vi "Main.vi"() -> ()   [LabVIEW 2020] (continued)
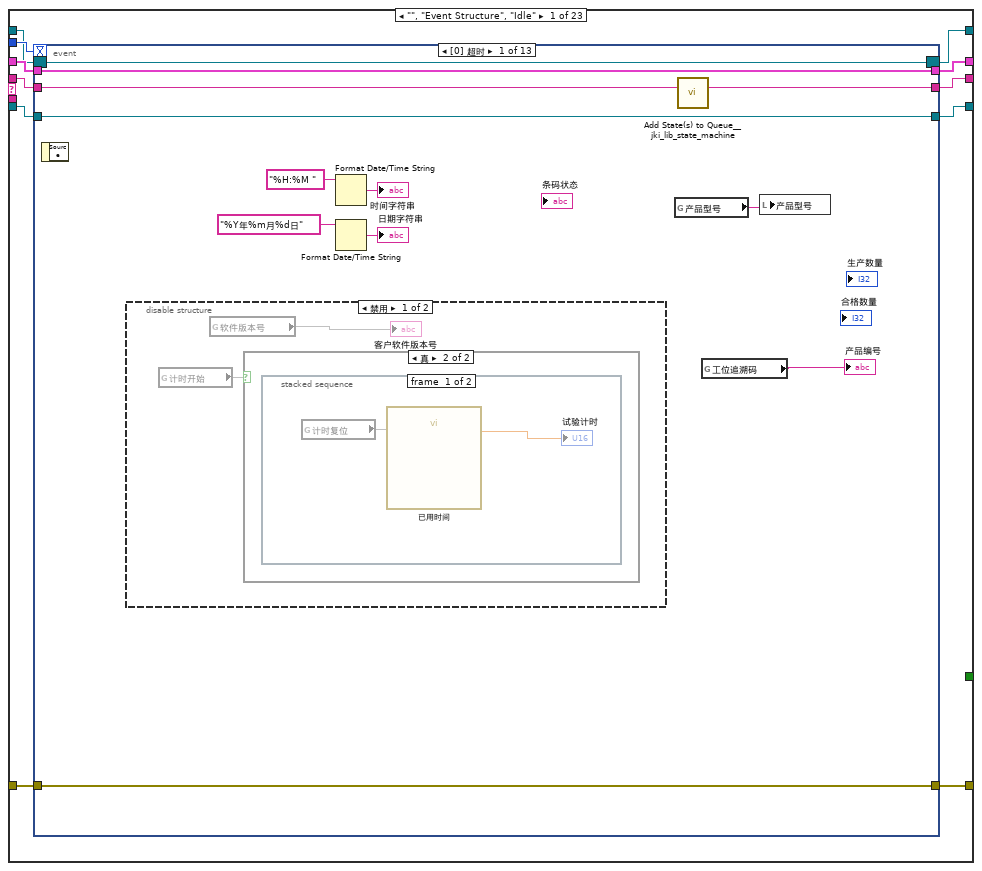
[diagram p2: hidden frame]
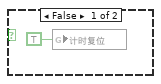
[diagram p3: hidden frame]
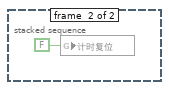
[diagram p4: hidden frame]
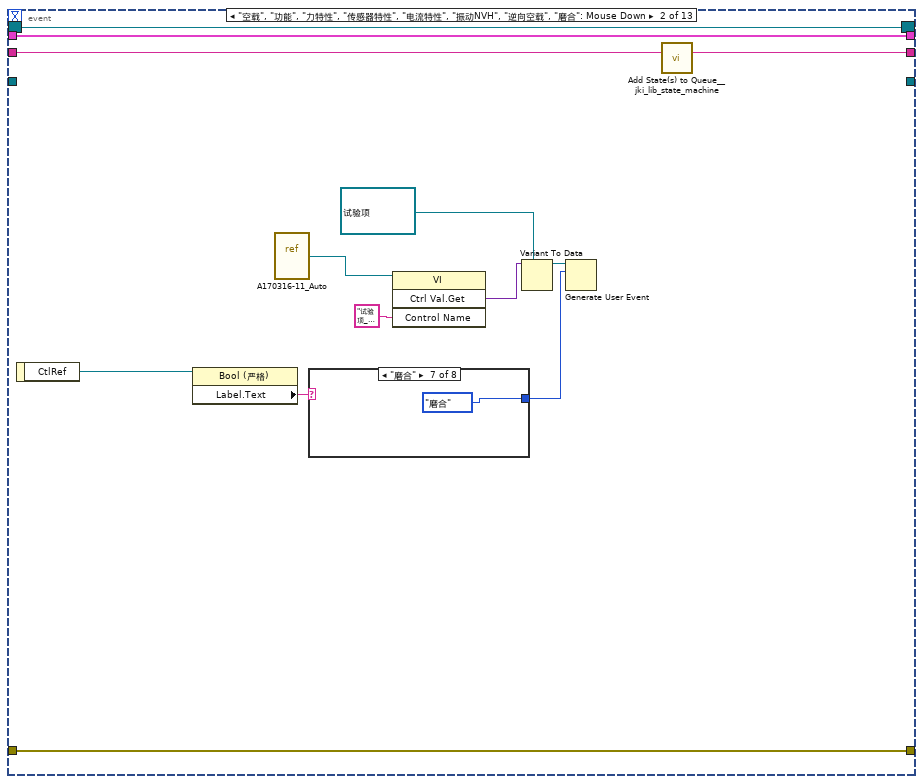
[diagram p6: hidden frame]
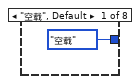
[diagram p7: hidden frame]
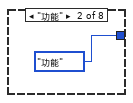
[diagram p8: hidden frame]
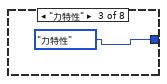
[diagram p9: hidden frame]
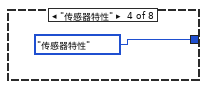
[diagram p10: hidden frame]
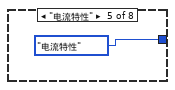
[diagram p11: hidden frame]
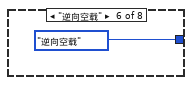
[diagram p12: hidden frame]
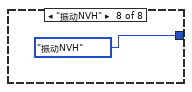
[diagram p13: hidden frame]
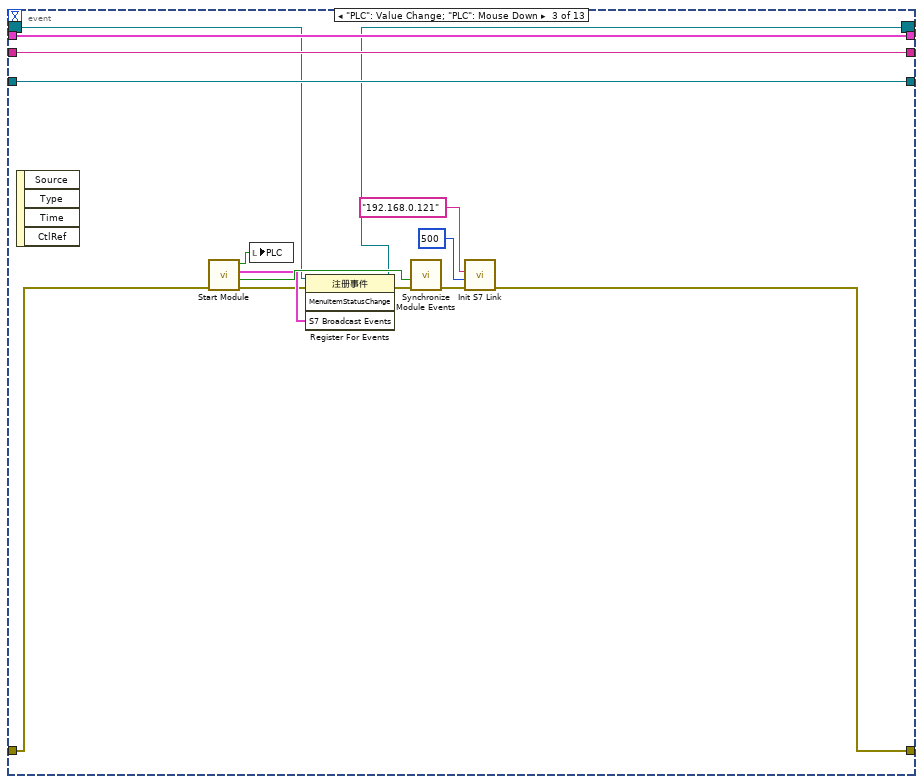
[diagram p14: hidden frame]
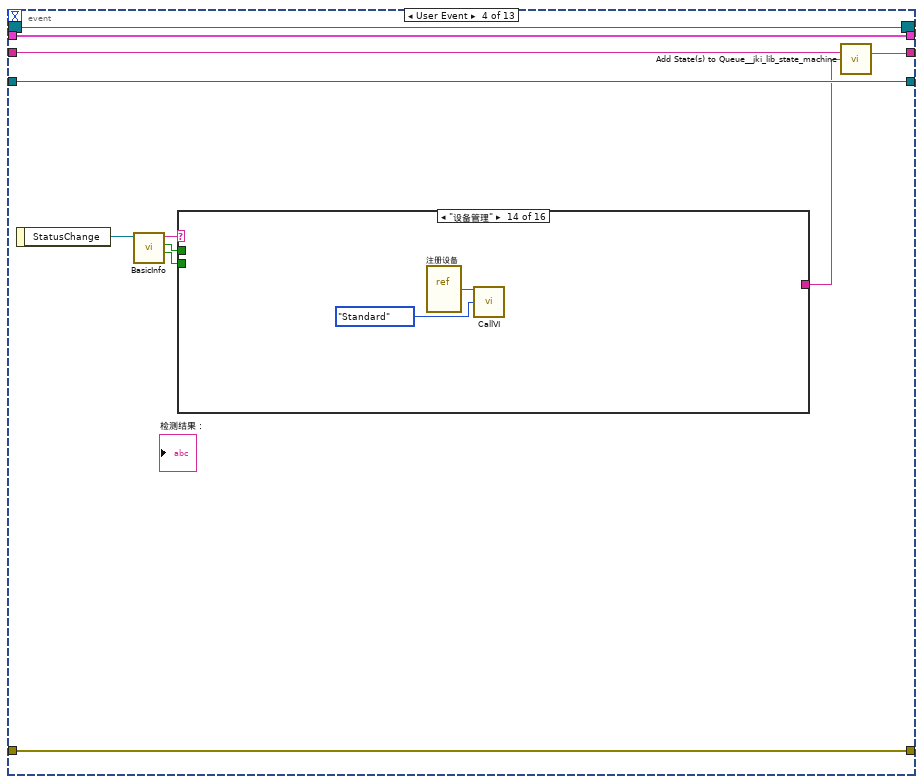
[diagram p15: hidden frame]
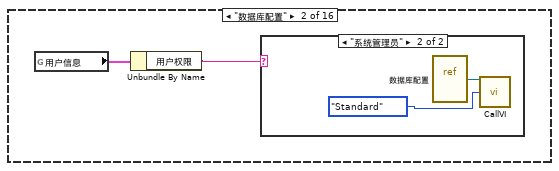
[diagram p17: hidden frame]
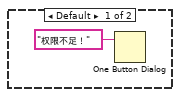
[diagram p18: hidden frame]
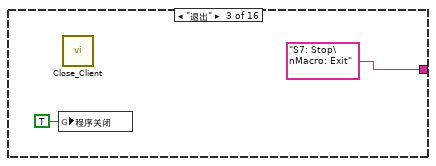
[diagram p19: hidden frame]
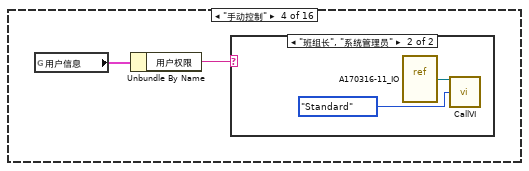
[diagram p20: hidden frame]
                  }
                }
              }
              frame True {
                n122 = Two Button Dialog(message="确定要退出自动？" ("消息")) -> (T button?=w202:bool)  [unwired: 2 in]
                n123 = case shown="真" w202 {
                  frame False {
                  }
                  frame True {
                    n124 = vi-ref "A170316-11_Auto.vi"() -> (w206:refnum<vi>)
                    n125 = invoke class="VI" method="Ctrl Val.Set"(reference=w206, "Control Name"="STEP" ("控件名"), "Value"="退出自动" ("控件名")) -> ()  [unwired: 2 in, 5 out]
                  }
                }
              }
            }
            n126 = call <vilib>:"Add State(s) to Queue__jki_lib_state_machine.vi"("State(s) in (\"\")"=w193) -> ("States Out"=w194:string)  [unwired: 14 in]
          }
          event "错误": Mouse Down {
            n127 = event-data() -> ()  [unwired: 1 in, 8 out]
            n128 = vi-ref "报警信息.vi"() -> (w209:refnum<vi>)
            n129 = call "CallVI.vi"("VI引用"=w209, "状态"=T3."Standard") -> ()  [unwired: 11 in, 3 out]
            n130 = call <vilib>:"Add State(s) to Queue__jki_lib_state_machine.vi"("State(s) in (\"\")"=w211) -> ("States Out"=w212:string)  [unwired: 14 in]
          }
          event Panel Close? {
            n131 = event-data() -> ()  [unwired: 1 in, 1 out]
            n132 = disable-structure shown="禁用" {
              frame Disabled {
                n133 = call "Close.vi"() -> ()  [unwired: 11 in, 1 out]
              }
              frame Enabled {
              }
            }
            n134 = global write "Global.vi" "程序关闭"(TRUE ("程序关闭")) -> ()
            n135 = call <vilib>:"Add State(s) to Queue__jki_lib_state_machine.vi"("State(s) in Front (\"\")"="S7: Stop\nMacro: Exit", "State(s) in (\"\")"=w221) -> ("States Out"=w220:string)  [unwired: 13 in]
            n136 = event-data("Discard?"=TRUE) -> ()  [unwired: 1 in, 1 out]
          }
          event "更换产品": Value Change {
            n137 = event-data() -> ("NewVal"=w224:refnum<vi>)  [unwired: 1 in, 5 out]
            n138 = stacked-sequence {
              tunnel: w224 -> [w230]
              tunnel: [w229] -> w222
              frame #0 {
                n139 = stacked-sequence {
                  tunnel: w230 -> [w231 _ _]
                  tunnel: [_ w242 _] -> w229
                  frame #0 {
                    n140 = disable-structure shown="禁用" {
                      frame Disabled {
                        n141 = vi-ref "Auto.vi"() -> (w238:refnum<vi>)
                        n142 = invoke class="VI" method="Ctrl Val.Get"(reference=w238, "Control Name"="产品_EVENT" ("控件名")) -> ("Get Control Value Variant"=w237:variant)  [unwired: 2 in, 3 out]
                        n143 = global read "Global.vi" "产品型号"() -> (w233:string)
                        n144 = local write "产品型号"(w233) -> ()
                        n145 = Variant To Data(type=refnum<user-event> refnum ("产品_EVENT"), Variant=w237) -> (data=w234:refnum<user-event>, error out=w232:errorcluster)  [unwired: 1 in]
                        n146 = Generate User Event(user event=w234, event data cluster=w233, error in=w232) -> ()  [unwired: 1 in, 2 out]
                      }
                      frame Enabled {
                      }
                    }
                    n147 = disable-structure shown="禁用" {
                      disable-tunnel: w231 -> [w240 _]
                      frame Disabled {
                        n148 = control-ref of="子面板"() -> (w239:refnum<vi>)
                        n149 = call "Call_SubPanal.vi"("VI引用句柄"=w240, "SubPnl引用句柄"=w239) -> ()  [unwired: 9 in, 1 out]
                      }
                      frame Enabled {
                      }
                    }
                  }
                  frame #1 {
                    n150 = global read "Global.vi" "启用CAN"() -> (w241:bool)
                    n151 = case shown="假" w241 {
                      tunnel: ["CAN: Stop" "CAN: Stop"] -> w242
                      frame False {
                      }
                      frame True {
                        (unwired) "CAN: Stop\nIdle\nCAN: Start"
                      }
                    }
                  }
                  frame #2 {
                    n152 = disable-structure shown="禁用" {
                      frame Disabled {
                        n153 = control-ref of="磨合"() -> (w245:refnum<vi>)
                        n154 = control-ref of="空载"() -> (w250:refnum<vi>)
                        n155 = control-ref of="功能"() -> (w251:refnum<vi>)
                        n156 = control-ref of="力特性"() -> (w252:refnum<vi>)
                        n157 = control-ref of="电流特性"() -> (w249:refnum<vi>)
                        n158 = control-ref of="传感器特性"() -> (w248:refnum<vi>)
                        n159 = control-ref of="逆向空载"() -> (w247:refnum<vi>)
                        n160 = control-ref of="振动NVH"() -> (w246:refnum<vi>)
                        n161 = global read "Global.vi" "试验项目"() -> (w255)
                        n162 = Build Array(w250, w251, w252, w249, w248, w247, w246, w245) -> (w254:refnum<vi>[])
                        n163 = for {
                          tunnel: w254 -> [w259] mode=indexing
                          tunnel: w255 -> [w260]
                          shift-right: [w256] -> _
                          shift-left: 2095 -> [w257]
                          i -> [w258]
                          n164 = case shown="真" w260 {
                            tunnel: w259 -> [w261 w269]
                            tunnel: w258 -> [_ _]
                            tunnel: w257 -> [w263 w266]
                            tunnel: [w263 w264] -> w256
                            frame False {
                              n165 = property class="Bool (严格)"(reference=w261, "Top"=2000) -> ()  [unwired: 1 in, 2 out]
                            }
                            frame True {
                              n166 = Add(x=w266, y=115) -> (x+y=w264:i32)
                              n167 = Bundle(w264, 1300) -> (w267:cluster{i32, i32})  [unwired: 1 in]
                              n168 = property class="Bool (严格)"(reference=w269, "Position"=w267) -> ()  [unwired: 1 in, 2 out]
                            }
                          }
                        }
                      }
                      frame Enabled {
                      }
                    }
                  }
                }
              }
            }
            n169 = call <vilib>:"Add State(s) to Queue__jki_lib_state_machine.vi"("State(s) in Front (\"\")"=w222, "State(s) in (\"\")"=w225) -> ("States Out"=w226:string)  [unwired: 13 in]
          }
          event "Andon": Value Change {
            w280 = "GP12终检" ("设备名称")
            n170 = event-data() -> ("NewVal"=w271:enum32{"未选择", "缺料报警", "质量报警", "故障报警"})  [unwired: 1 in]
            n171 = global read "Global1.vi" "用户信息"() -> (w270:T6)
            n172 = Unbundle By Name(w270) -> ("用户权限"=w279:string)
            n173 = case shown="\"故障报警\"" w271 {
              tunnel: w280 -> [_ _ _ _]
              tunnel: w279 -> [_ _ _ _]
              tunnel: [enum16{"设备离线", "设备正常", "设备缺料", "设备故障", "质量报警"}."设备正常" ("设备状态") enum16{"设备离线", "设备正常", "设备缺料", "设备故障", "质量报警"}."设备缺料" ("设备状态") enum16{"设备离线", "设备正常", "设备缺料", "设备故障", "质量报警"}."质量报警" ("设备状态") enum16{"设备离线", "设备正常", "设备缺料", "设备故障", "质量报警"}."设备故障" ("设备状态")] -> w277
              frame "未选择", Default {
              }
              frame "缺料报警" {
              }
              frame "质量报警" {
              }
              frame "故障报警" {
              }
            }
            n174 = Bundle By Name(cluster=T4 {"设备名称"="", "操作人员"="", "设备状态"=enum."设备离线", "附加信息"=""} ("设备信息"), "设备名称"=w280, "操作人员"=w279, "设备状态"=w277) -> (w272:T4)
            n175 = call "Change_Client.vi"("设备信息"=w272) -> ()  [unwired: 10 in, 1 out]
          }
        }
      }
      frame "---------- Core ----------" {
        n176 = call <vilib>:"Add State(s) to Queue__jki_lib_state_machine.vi"("State(s) in (\"\")"=w290) -> ("States Out"=w289:string)  [unwired: 14 in]
      }
      frame Default {
        w302 = 42 items=["No error", "Argument error", "Memory is full", "Out of zone", "End of file", "File already open", "Generic file I/O error", "File not found", "File permission error", "Disk is full", "Duplicate path", "Too many files open", "System feature not enabled", "Resource file not found", "Cannot add resource", "Resource not found", "Image not found", "Image memory error", "Pen does not exist", "Config type invalid", "Config token not found", "Config parse error", "Config memory error", "Bad external code format", "Bad external code offset", "External code not present", "Null window", "Destroy window error", "Null menu", "Print aborted", "Bad print record", "Print driver error", "Windows error during printing", "Memory error during printing", "Print dialog error", "Generic print error", "Invalid device refnum", "Device not found", "Device parameter error", "Device unit error", "Cannot open device", "Device call aborted", "Generic error", "Cancelled by user", "Object ID too low", "Object ID too high", "Object not in heap", "Unknown heap", "Unknown object (invalid DefProc)", "Unknown object (DefProc not in table)", "Message out of range", "Invalid (null) method", "Unknown message", "Manager call not supported", "Bad address", "Network operation in progress", "Network operation timed out", "Connection is busy", "Network attribute not supported", "Network error", "Address in use", "System out of memory", "Connection aborted", "Connection refused", "Not connected", "Already connected", "Connection closed", "Initialization error (interapplication manager)", "Bad occurrence", "Wait on unbound occurrence handler", "Occurrence queue overflow", "Datalog type conflict", "Unused", "Unrecognized type (interapplication manager)", "Memory corrupt", "Failed to make temporary DLL", "Old CIN version", "Drag socket not found", "Failed to load drop-object", "Failed to register OLE object", "Failed to release OLE object", "Format specifier type mismatch", "Unknown format specifier", "Too few format specifiers", "Too many format specifiers", "Scan failed", "Newer CIN version", "Error converting to variant", "Runtime menu error", "Password tampered", "Variant attribute not found", "Incompatible variant data type", "Event data is not available", "Event Store is not present", "Occurrence is not found", "Event Queue is not created", "Event info is not available", "Refnum passed is NULL", "Error retrieving Class GUID", "Error retrieving CoClass GUID", "Error retrieving TypeLib GUID.", "Bad built application magic bytes.", "Specific driver is different from the specific driver associated with the Logical Name.", "There is no session opened to the class driver.", "Max Error", "MAX - Error with config objects", "MAX - Error loading configuration", "MAX - Group not supported"]
        # "Current State"
        n177 = Format Into String(format string="Software Exception: Unhandled State \"%s\"." ("message"), error in=w298, w293) -> (resulting string=w301:string, error out=w300:errorcluster)  [unwired: 1 in]
        n178 = call <vilib>:"Error Cluster From Error Code.vi"("show call chain? (False)"=TRUE, "error in (no error)"=w300, "error message (\"\")"=w301, "error code (0)"=w302) -> ("error out"=w299:errorcluster)  [unwired: 5 in]
        n179 = call <vilib>:"Add State(s) to Queue__jki_lib_state_machine.vi"("State(s) in (\"\")"=w297) -> ("States Out"=w296:string)  [unwired: 14 in]
      }
      frame "Initialize Core Data" {
        # "originally closed?"
        # "exe?"
        n180 = property class="VI"() -> ("Front Panel.Open"=w313:bool)  [unwired: 2 in, 2 out]
        n181 = property class="App"() -> ("App.Kind"=w312:T5)  [unwired: 2 in, 2 out]
        n182 = control-ref of="Current VI Reference"() -> (w306:refnum<vi>)
        n183 = Not(x=w313) -> (.not. x?=w310:bool)
        n184 = Equal?(x=w312, y=T5."Run Time System" ("Application:Kind")) -> (x = y?=w309:bool)
        n185 = Or(x=w310, y=w309) -> (x .or. y?=w307:bool)
        n186 = Bundle By Name(cluster=w308, "Core.Current VI Reference"=w306, "Core.Close Panel on Exit?"=w307) -> (w315:T7)
        n187 = call <vilib>:"Add State(s) to Queue__jki_lib_state_machine.vi"("State(s) in (\"\")"=w317) -> ("States Out"=w316:string)  [unwired: 14 in]
      }
      frame "Error Handler" {
        n188 = call <vilib>:"General Error Handler.vi"("error in (no error)"=w321) -> ()  [unwired: 10 in, 5 out]
        n189 = call <vilib>:"Add State(s) to Queue__jki_lib_state_machine.vi"("State(s) in Front (\"\")"="/* Post Error States", "State(s) in (\"\")"=w325) -> ("States Out"=w324:string)  [unwired: 13 in]
      }
      frame "Exit" {
        n190 = Quit LabVIEW(quit? (T)=TRUE ("退出？(T)")) -> ()
        n191 = call <vilib>:"Add State(s) to Queue__jki_lib_state_machine.vi"("State(s) in (\"\")"=w333) -> ("States Out"=w332:string)  [unwired: 14 in]
      }
      frame "--------- Library --------" {
        n192 = call <vilib>:"Add State(s) to Queue__jki_lib_state_machine.vi"("State(s) in (\"\")"=w339) -> ("States Out"=w338:string)  [unwired: 14 in]
      }
      frame "S7: Initialize" {
        n193 = property on="PLC" class="Bool (严格)"("Val(Sgnl)"=FALSE ("值(信号)")) -> ()  [unwired: 2 in, 2 out]
      }
      frame "S7: Stop" {
        n194 = call "Stop Module.vi"("error in (no error)"=w348) -> ("error out"=w347:errorcluster)  [unwired: 10 in]
        n195 = call <vilib>:"Add State(s) to Queue__jki_lib_state_machine.vi"("State(s) in (\"\")"=w349) -> ("States Out"=w350:string)  [unwired: 14 in]
      }
      frame "CAN: Start" {
        n196 = call <vilib>:"Add State(s) to Queue__jki_lib_state_machine.vi"("State(s) in (\"\")"=w355) -> ("States Out"=w356:string)  [unwired: 14 in]
      }
      frame "CAN: Stop" {
        n197 = call <vilib>:"Add State(s) to Queue__jki_lib_state_machine.vi"("State(s) in (\"\")"=w361) -> ("States Out"=w362:string)  [unwired: 14 in]
      }
      frame "---------- Data ----------" {
        n198 = call <vilib>:"Add State(s) to Queue__jki_lib_state_machine.vi"("State(s) in (\"\")"=w370) -> ("States Out"=w369:string)  [unwired: 14 in]
      }
      frame "Data: Initialize" {
        (unwired) FALSE ("计时结束")
        w374 = T8 {"Current VI Reference"=refnum, "Close Panel on Exit?"=FALSE}  # Core
        w376 = TRUE  # Your Boolean data
        w375 = ""  # Your string data
        n199 = global write "Global.vi" "程序关闭"(FALSE ("程序关闭")) -> ()
        n200 = Bundle("Core"=w374, "Your Boolean data"=w376, "Your string data"=w375) -> (w378:T7)  [unwired: 1 in]
        n201 = call <vilib>:"Add State(s) to Queue__jki_lib_state_machine.vi"("State(s) in (\"\")"=w380) -> ("States Out"=w379:string)  [unwired: 14 in]
      }
      frame "Data: Cleanup" {
        n202 = Unbundle By Name(w383) -> ("Core.Current VI Reference"=w386:refnum<vi>)
        n203 = Close Reference(reference=w386, error in (no error)=w385) -> (error out=w384:errorcluster)
        n204 = call <vilib>:"Add State(s) to Queue__jki_lib_state_machine.vi"("State(s) in (\"\")"=w388) -> ("States Out"=w387:string)  [unwired: 14 in]
      }
      frame "---------- UI ----------" {
        # "Do not put any code in this frame.\n(It is a separator no-op. You can make a copy of this frame to create a new UI frame)"
        n205 = call <vilib>:"Add State(s) to Queue__jki_lib_state_machine.vi"("State(s) in (\"\")"=w394) -> ("States Out"=w393:string)  [unwired: 14 in]
      }
      frame "UI: Initialize" {
        n206 = disable-structure shown="启用" {
          disable-tunnel: [w408 _] -> w398
          disable-tunnel: w395 -> [w406 _]
          frame Enabled {
            n207 = vi-ref "A170316-11_Auto.vi"() -> (w407:refnum<vi>)
            n208 = property class="VI"(reference=w407) -> (reference out=w405:refnum<vi>, "FP.State"=w404:T3)  [unwired: 1 in, 1 out]
            n209 = case shown="\"Invalid\", \"Closed\"" w404 {
              tunnel: w406 -> [w414 w416]
              tunnel: w405 -> [w415 w417]
              tunnel: [w413 w417] -> w402
              tunnel: [w412 w416] -> w403
              frame "Standard", Default {
                n210 = invoke class="VI" method="FP.Close"(reference=w415, error in=w414) -> (reference out=w413:refnum<vi>, error out=w412:errorcluster)  [unwired: 1 in, 1 out]
              }
              frame "Invalid", "Closed" {
              }
            }
            n211 = invoke on="子面板" class="SubPnl" method="Insert VI"(error in=w403, "VI Ref"=w402) -> (error out=w411:errorcluster)  [unwired: 2 in, 3 out]
            n212 = invoke class="VI" method="Run VI"(reference=w402, error in=w411, "Wait until done"=FALSE ("结束前等待"), "Auto Dispose Ref"=TRUE ("自动销毁引用")) -> (error out=w408:errorcluster)  [unwired: 1 in, 4 out]
          }
          frame Disabled {
            n213 = vi-ref "Auto.vi"() -> (w419:refnum<vi>)
            n214 = call "CallVI.vi"("VI引用"=w419, "状态"=T3."Maximized") -> ()  [unwired: 11 in, 3 out]
          }
        }
        n215 = call <vilib>:"Add State(s) to Queue__jki_lib_state_machine.vi"("State(s) in (\"\")"=w401) -> ("States Out"=w400:string)  [unwired: 14 in]
      }
      frame "UI: Init" {
        n216 = stacked-sequence {
          tunnel: w421 -> [_ _ _ _ _]
          frame #0 {
            n217 = disable-structure shown="启用" {
              frame Disabled {
                n218 = call "Open.vi"() -> ()  [unwired: 11 in, 1 out]
              }
              frame Enabled {
              }
            }
          }
          frame #1 {
            n219 = global write "Global.vi" "程序关闭"(FALSE ("程序关闭")) -> ()
          }
          frame #2 {
            n220 = shared-variable "我的电脑\\Global.lvlib\\总成追溯码"("   " ("工位追溯码")) -> ()  [unwired: 1 in, 1 out]
            n221 = global read "Global1.vi" "用户信息"() -> (w430:T6)
            n222 = global read "Global1.vi" "联机模式"() -> (w427:enum16{"单机", "联网"})
            n223 = Unbundle By Name(w430) -> ("用户名"=→"userName":string, "用户权限"=→"userStatus":string)
            n224 = case shown="\"单机\", 默认" w427 {
              tunnel: ["联网" ("connectionMode") "单机" ("connectionMode")] -> w433
              frame "联网" {
              }
              frame "单机", Default {
              }
            }
            "connectionMode" <- w433
            "产品型号" <- "" ("产品型号")
          }
          frame #3 {
            n225 = control-ref of="提示信息"() -> (w439:refnum<vi>)
            n226 = control-ref of="自动"() -> (w440:refnum<vi>)
            n227 = control-ref of="错误"() -> (w441:refnum<vi>)
            n228 = control-ref of="Result"() -> (w442:refnum<vi>)
            n229 = control-ref of="更换产品"() -> (w438:refnum<vi>)
            n230 = global write "Global.vi" "提示信息"(w439) -> ()
            n231 = global write "Global.vi" "程序自动"(w440) -> ()
            n232 = global write "Global.vi" "报警图标"(w441) -> ()
            n233 = global write "Global.vi" "Result"(w442) -> ()
            n234 = global write "Global.vi" "更换产品"(w438) -> ()
            n235 = control-ref of="条码状态"() -> (w437:refnum<vi>)
            n236 = control-ref of="检测结果："() -> (w436:refnum<vi>)
            n237 = global write "Global.vi" "条码状态"(w437) -> ()
            n238 = global write "Global.vi" "结果显示字"(w436) -> ()
          }
          frame #4 {
            n239 = global read "Global.vi" "Result"() -> (w445:refnum<vi>)
            n240 = property class="Tbl"(reference=w445, "Row Headers[]"=string[] [], "Value"=string[][] []) -> ()  [unwired: 1 in, 2 out]
            n241 = call "Start_Client.vi"() -> ()  [unwired: 12 in]
          }
        }
        n242 = call <vilib>:"Add State(s) to Queue__jki_lib_state_machine.vi"("State(s) in (\"\")"=w425) -> ("States Out"=w424:string)  [unwired: 14 in]
      }
      frame "UI: Config" {
        n243 = vi-ref "A170316-11_config.vi"() -> (w448:refnum<vi>)
        n244 = call "CallVI.vi"("VI引用"=w448, "状态"=T3."Standard") -> ()  [unwired: 11 in, 3 out]
        n245 = call <vilib>:"Add State(s) to Queue__jki_lib_state_machine.vi"("State(s) in (\"\")"=w453) -> ("States Out"=w452:string)  [unwired: 14 in]
      }
      frame "UI: Cursor Set" {
        # "Argument"
        n246 = case shown="\"Idle\", 默认" w456 {
          tunnel: w458 -> [w463 w465]
          tunnel: [w462 w464] -> w457
          frame "Idle", Default {
            n247 = call <vilib>:"Unset Busy.vi"("error in (no error)"=w463) -> ("error out"=w462:errorcluster)  [unwired: 10 in]
          }
          frame "Busy" {
            n248 = call <vilib>:"Set Busy.vi"("error in (no error)"=w465) -> ("error out"=w464:errorcluster)  [unwired: 9 in, 1 out]
          }
        }
        n249 = call <vilib>:"Add State(s) to Queue__jki_lib_state_machine.vi"("State(s) in (\"\")"=w461) -> ("States Out"=w460:string)  [unwired: 14 in]
      }
      frame "UI: Front Panel State" {
        # "Argument"
        n250 = Unbundle By Name(w470) -> ("Core.Current VI Reference"=w469:refnum<vi>)
        n251 = case shown="\"Open\", 默认" w468 {
          tunnel: w472 -> [w478 w491]
          tunnel: [w480 w492] -> w471
          tunnel: w469 -> [w479 w489]
          frame "Open", Default {
            n252 = property class="VI"(reference=w479, error in=w478) -> (reference out=w476:refnum<vi>, error out=w477:errorcluster, "Front Panel.Open"=w475:bool)
            n253 = case shown="假" w475 {
              tunnel: [w483 w486] -> w480
              tunnel: w477 -> [w482 w486]
              tunnel: w476 -> [w481 _]
              frame False {
                n254 = invoke class="VI" method="FP.Open"(reference=w481, error in=w482, "Activate"=TRUE, "State"=T3."Standard") -> (error out=w483:errorcluster)  [unwired: 1 in, 4 out]
              }
              frame True {
              }
            }
          }
          frame "Close" {
            n255 = property class="VI"(reference=w489, error in=w491) -> (reference out=w488:refnum<vi>, error out=w490:errorcluster, "Front Panel.Open"=w487:bool)
            n256 = case shown="真" w487 {
              tunnel: [w493 w496] -> w492
              tunnel: w490 -> [w493 w495]
              tunnel: w488 -> [_ w494]
              frame False {
              }
              frame True {
                n257 = invoke class="VI" method="FP.Close"(reference=w494, error in=w495) -> (error out=w496:errorcluster)  [unwired: 1 in, 2 out]
              }
            }
          }
        }
        n258 = call <vilib>:"Add State(s) to Queue__jki_lib_state_machine.vi"("State(s) in (\"\")"=w474) -> ("States Out"=w473:string)  [unwired: 14 in]
      }
      frame "---------- Macro ----------" {
        n259 = call <vilib>:"Add State(s) to Queue__jki_lib_state_machine.vi"("State(s) in (\"\")"=w502) -> ("States Out"=w501:string)  [unwired: 14 in]
      }
      frame "Macro: Initialize" {
        n260 = call <vilib>:"Add State(s) to Queue__jki_lib_state_machine.vi"("State(s) in Front (\"\")"="Data: Initialize\nInitialize Core Data\nS7: Initialize\nIdle\nUI: Init\nUI: Front Panel State >> Open\nUI: Initialize\nUI: Config", "State(s) in (\"\")"=w509) -> ("States Out"=w508:string)  [unwired: 13 in]
      }
      frame "Macro: Exit" {
        n261 = Unbundle By Name(w519) -> ("Core.Close Panel on Exit?"=w518:bool)
        n262 = Select(t="UI: Front Panel State >> Close", s=w518, f="") -> (s? t:f=w515:string)
        n263 = Quit LabVIEW(quit? (T)=TRUE ("退出？(T)")) -> ()
        n264 = call <vilib>:"Add State(s) to Queue__jki_lib_state_machine.vi"("State(s) in (\"\")"=w515, "State(s) at Back (\"\")"="Data: Cleanup\nExit") -> ("States Out"=w513:string)  [unwired: 13 in]
        n265 = call <vilib>:"Add State(s) to Queue__jki_lib_state_machine.vi"("State(s) in Front (\"\")"=w513, "State(s) in (\"\")"=w522) -> ("States Out"=w521:string)  [unwired: 13 in]
      }
    }
  }
  n266 = call-dynamic "Cleanup.vi"("MenuStrip in"=w6) -> ()  [unwired: 10 in, 1 out]
